vi "Basculas Fabela MultiController.vi"() -> ()   [LabVIEW 2019]
uses:
  <vilib>/Utility/file.llb/Read Delimited Spreadsheet (string).vi
  Subprogramas/Variable global de carga.vi
  <vilib>/Utility/file.llb/Write Delimited Spreadsheet (string).vi
  <vilib>/Utility/error.llb/Error Cluster From Error Code.vi
  <vilib>/ErrorRing/Error Ring.xnode
  <vilib>/Plasmionique/MB Master/MB_Master_Serial/MB_Master_Serial.lvclass
panel:
  in  "Secret button":bool
  out "ReportXlsxPath":path=path "C:/Temp/Basculas Fabela MultiController/Documentos/Reporte.txt"
  out "CtrlClusterOld":T1(array[cluster])
  out "CtrlNumberOld":i32
  in  "ConfChange":bool caption="Lectura de controladores"
  out "PythonPath":path=path "C:/Temp/Insagro/Documentos/TXTaXLSX.exe"
  out "ReportPath":path=path "C:/Temp/Basculas Fabela MultiController/Documentos/Reporte.txt"
  out "ComNumberPath":path=path "C:/Temp/Basculas Fabela MultiController/Documentos/ComNumber.txt"
  out "ComConfigPath":path=path "C:/Temp/Basculas Fabela MultiController/Documentos/ComConfig.txt"
  out "TxtPath":path=path "C:/Temp/Basculas Fabela MultiController/Documentos/Recetas.txt"
  out "Tabs":enum32{"Home", "Main", "Setup"}(tab)=enum."Setup"
  in  "Controllers Load":T2(array[cluster])=[{"ControlerNum"="Controlador 1", "Recipe"="", "Status"=9868950}] caption="Controladores"
  in  "Carga total":bool
  out "Main Load":enum32{"No load", "Load"}(tab)
  out "Ring 2":u16(ring)
  in  "Read":bool caption="Lectura de controladores"
  out "Loading Text":string
  out "TABLA DE RECETAS":string[][](table)
  in  "SecretAnimationCtrl":i32=1 caption="Selección de animación secreta" min=1
  in  "Array CtrlCluster":T1(array[cluster])=[{"Control#"="Control 1", "Com"=""}]
  in  "CtrlNumber":i32=1 caption="Número de controladores" min=1
  in  "Boton Guardar Cambios":bool
  in  "Settings Nav Button":bool=TRUE
  in  "Recetas Nav Button":bool
  in  "Home Nav Button":bool
  # "Seleccione en cada pantalla la fórmula que desee servir"
  # "Peso Objetivo"
  # "Número de Fórmula"
  # "Peso Servido"
  # "Tolva 1"
  # "Tolva 2"
  # "Tolva 3"
  # "Tolva 4"
  # "Indicador Báscula Sirviendo"
  # "Botón Ajuste Manual"
  # "Indicador Falta Material"
  # "FORMULA SELECCIONADA"
  # "CONFIGURACION DE COMUNICACION"
  # "Seleccione los puertos de comunicación"
  # "Controladores"
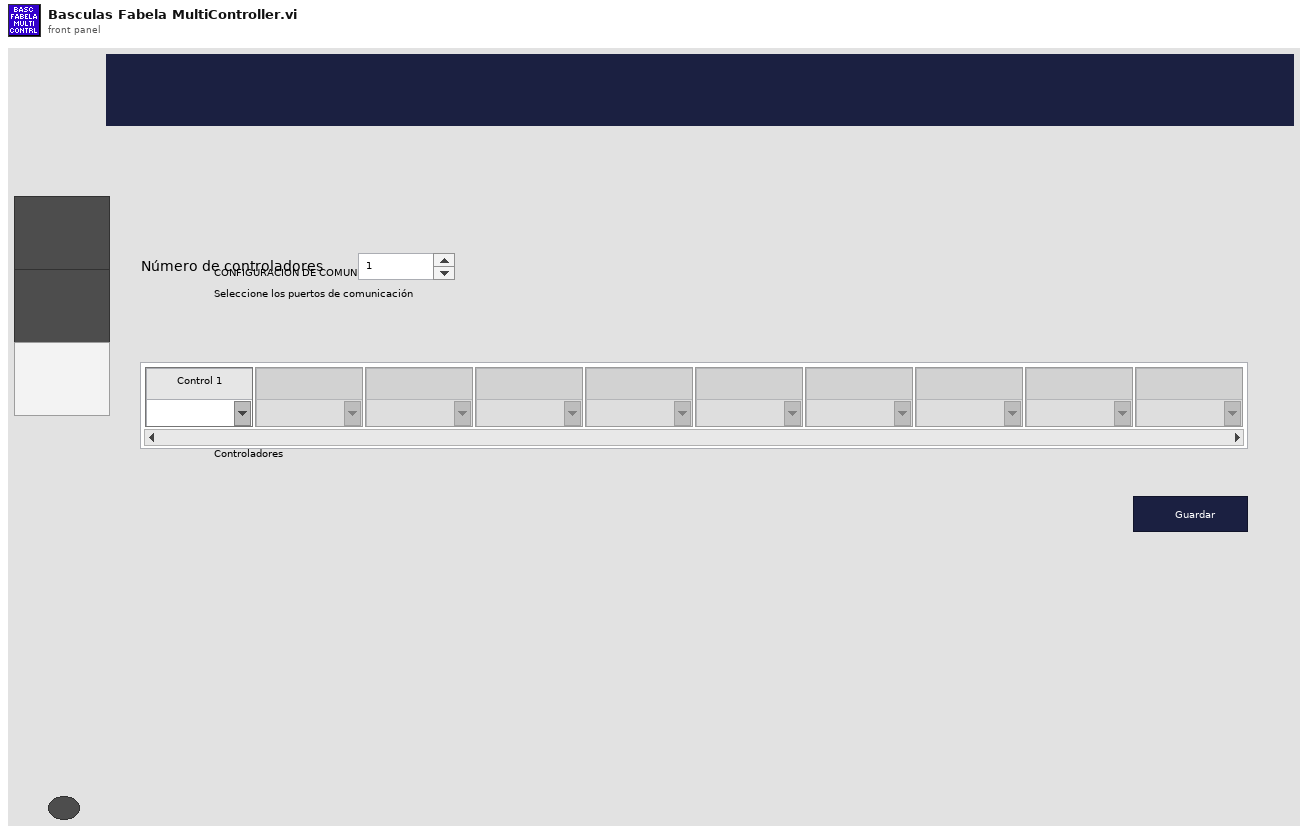
[diagram p1: front panel]
types:
  T1 = cluster{"Control#":string, "Com":refnum<visa-resource-name>}[]
  T2 = cluster{"ControlerNum":string, "Recipe":string, "Status":u32}[]
  T3 = enum8{"Enabled", "Disabled", "Disabled and Grayed Out"}
  T4 = cluster{"Control#":string, "Com":refnum<visa-resource-name>}
  T5 = cluster{"ControlerNum":string, "Recipe":string, "Status":u32}
  T6 = typedef "Control 2.ctl" = refnum<class "MB_Master_Serial.lvclass">[]
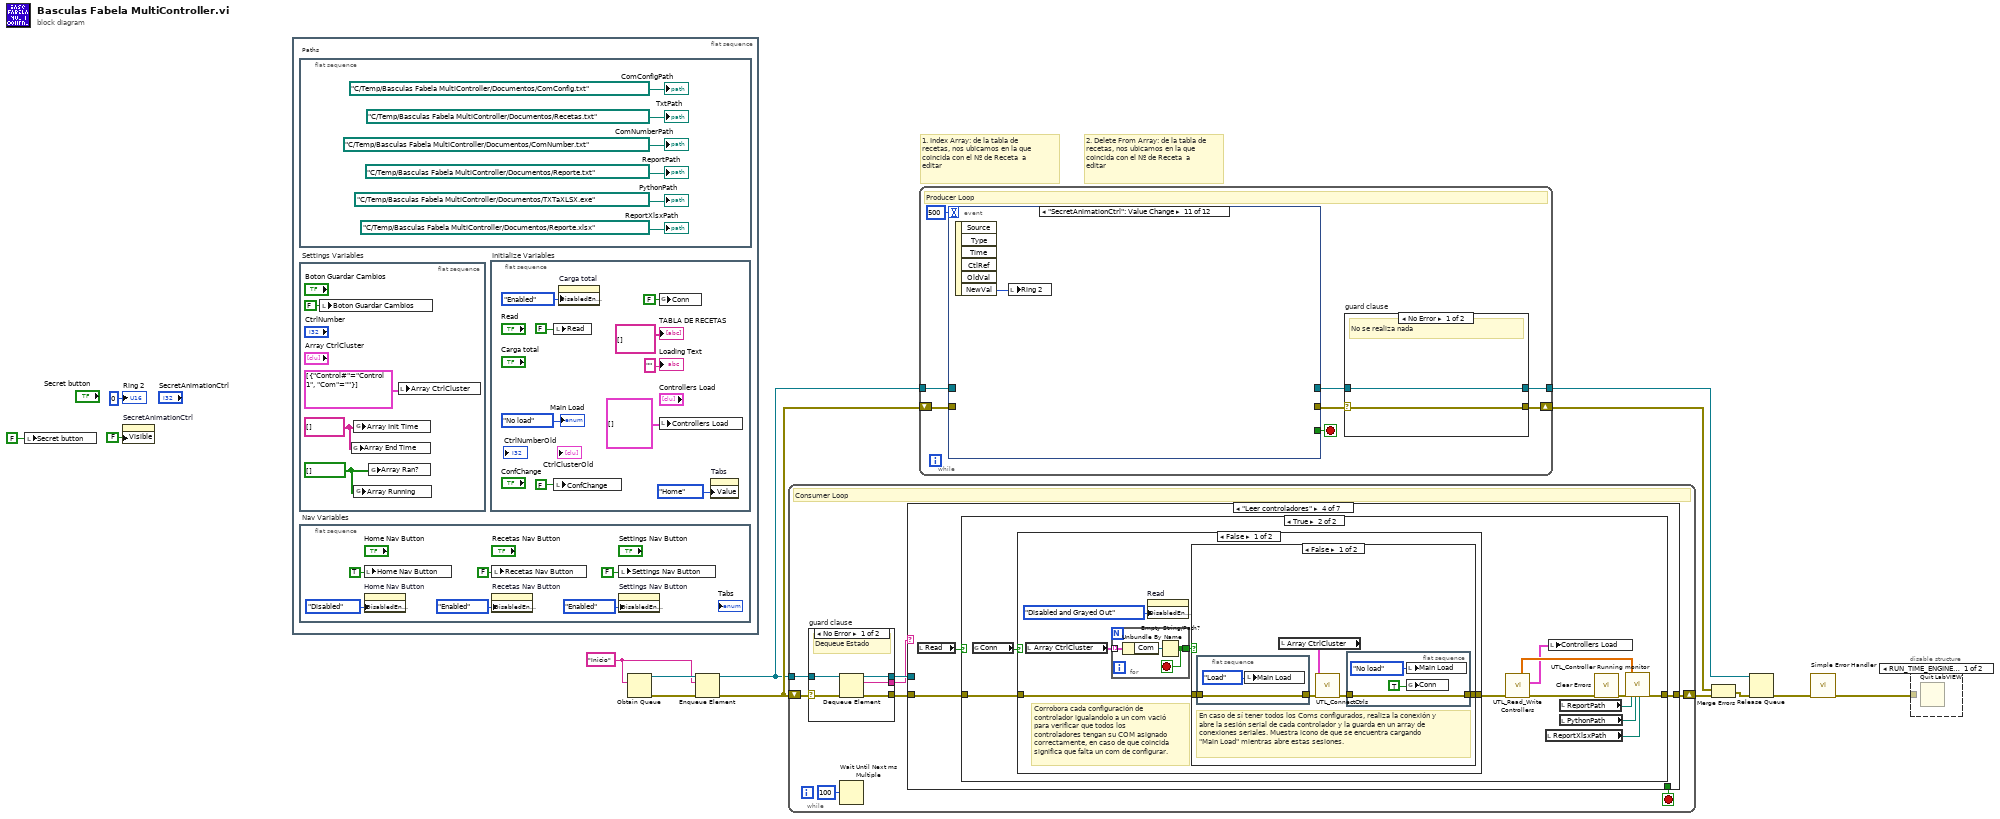
[diagram p0: block diagram]
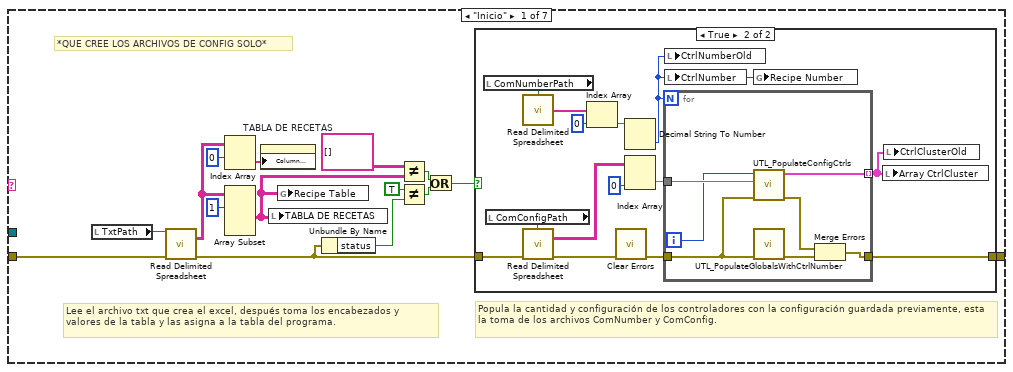
[diagram p2: hidden frame]
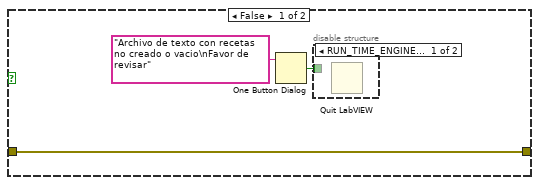
[diagram p3: hidden frame]
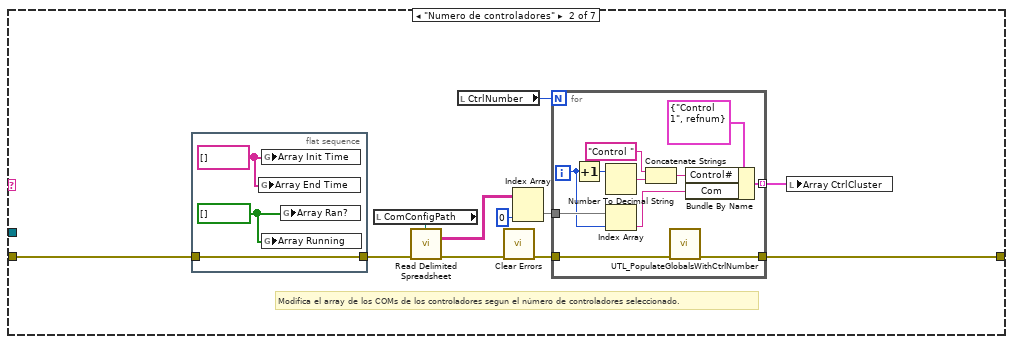
[diagram p5: hidden frame]
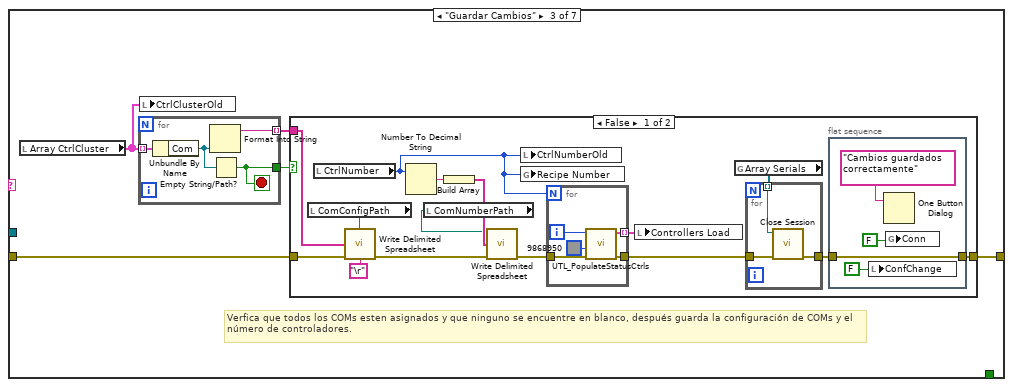
[diagram p6: hidden frame]
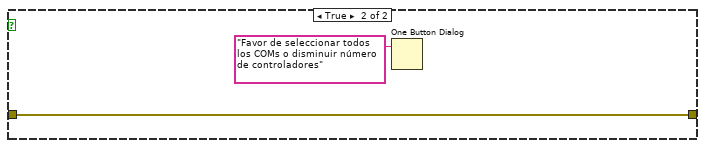
[diagram p7: hidden frame]
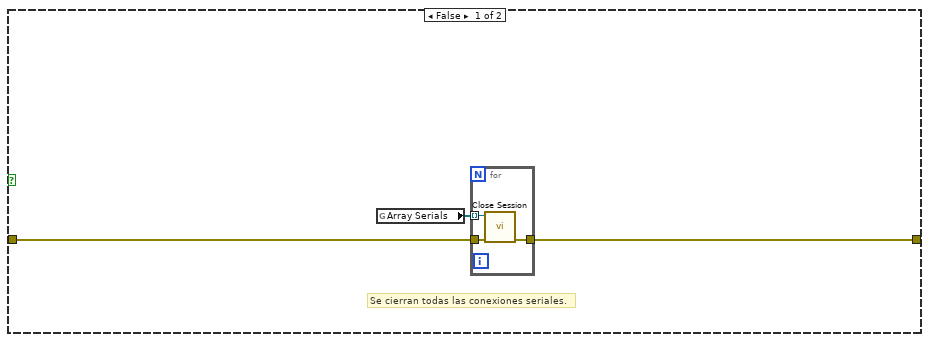
[diagram p8: hidden frame]
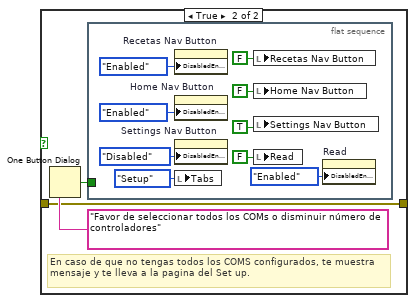
[diagram p9: hidden frame]
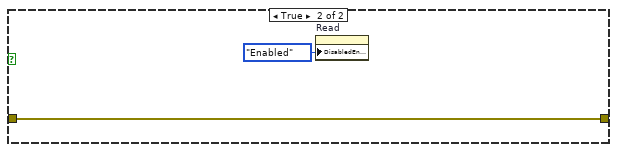
[diagram p10: hidden frame]
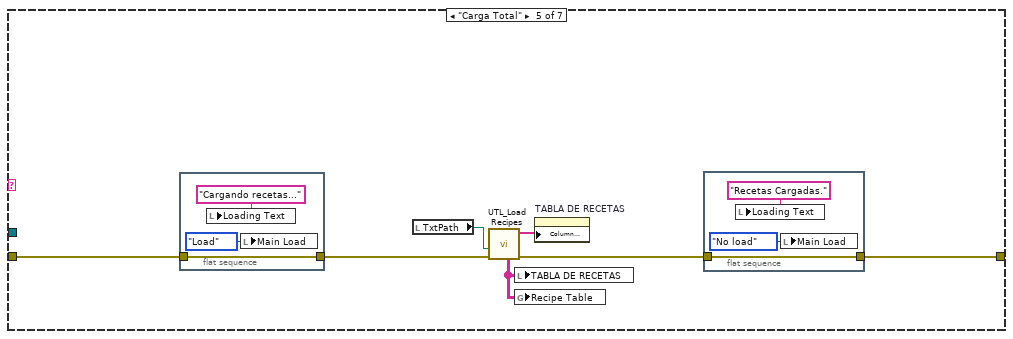
[diagram p11: hidden frame]
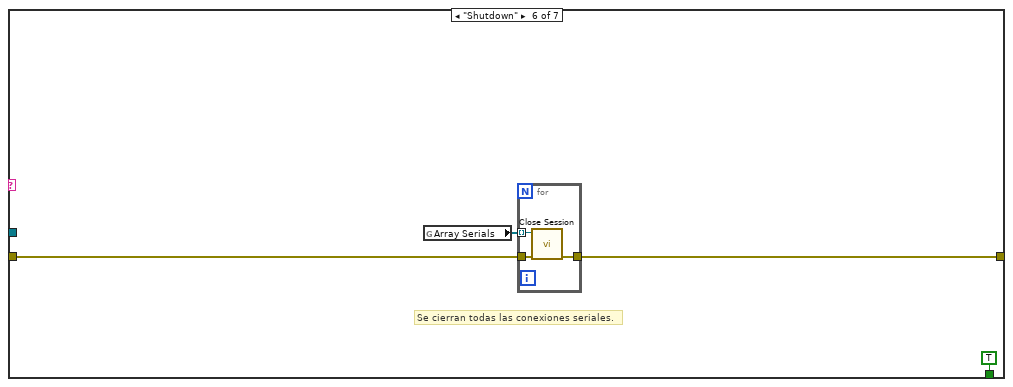
[diagram p12: hidden frame]
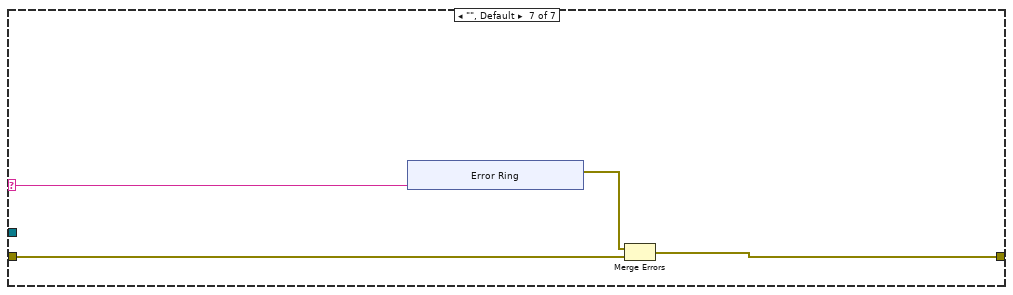
[diagram p13: hidden frame]
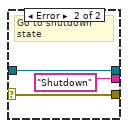
[diagram p14: hidden frame]
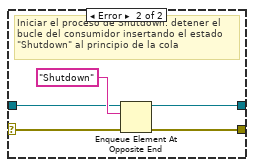
[diagram p15: hidden frame]
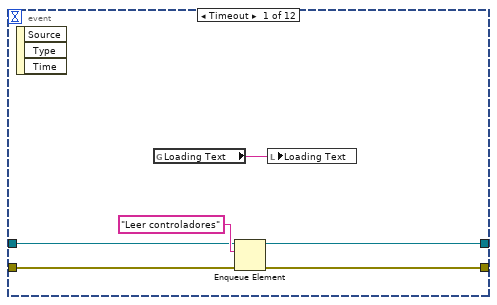
[diagram p16: hidden frame]
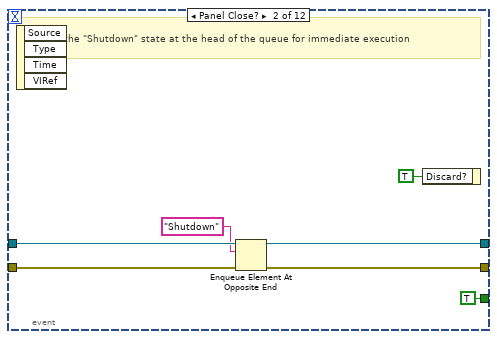
[diagram p17: hidden frame]
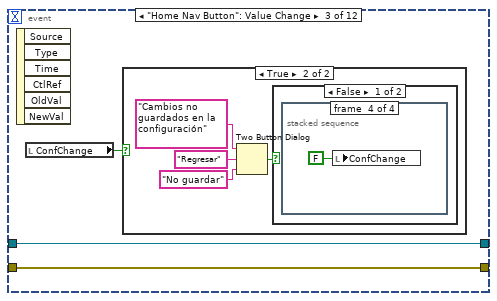
[diagram p18: hidden frame]
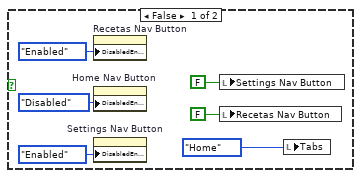
[diagram p19: hidden frame]
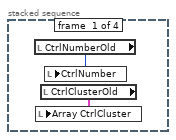
[diagram p20: hidden frame]
diagram:
  w5 = "Inicio"
  # "2. Delete From Array: de la tabla de recetas, nos ubicamos en la que coincida con el Nº de Receta  a editar"
  # "1. Index Array: de la tabla de recetas, nos ubicamos en la que coincida con el Nº de Receta  a editar"
  n1 = local write "Secret button"(FALSE ("Secret button")) -> ()
  n2 = property on="SecretAnimationCtrl" class="DigNum (strict)"("Visible"=FALSE) -> ()  [unwired: 2 in, 2 out]
  n3 = flat-sequence {
    frame #0 {
      # "Initialize Variables"
      # "Nav Variables"
      # "Paths"
      # "Settings Variables"
      n4 = flat-sequence {
        frame #0 {
          "TxtPath" <- path "C:/Temp/Basculas Fabela MultiController/Documentos/Recetas.txt" ("name or relative path")
          "ComConfigPath" <- path "C:/Temp/Basculas Fabela MultiController/Documentos/ComConfig.txt" ("name or relative path")
          "ComNumberPath" <- path "C:/Temp/Basculas Fabela MultiController/Documentos/ComNumber.txt" ("name or relative path")
          "ReportPath" <- path "C:/Temp/Basculas Fabela MultiController/Documentos/Reporte.txt" ("name or relative path")
          "PythonPath" <- path "C:/Temp/Basculas Fabela MultiController/Documentos/TXTaXLSX.exe" ("name or relative path")
          "ReportXlsxPath" <- path "C:/Temp/Basculas Fabela MultiController/Documentos/Reporte.xlsx" ("name or relative path")
        }
      }
      n5 = flat-sequence {
        frame #0 {
          w38 = bool[] [] ("Array Ran?")
          w37 = string[] [] ("Array Init Time")
          n6 = local write "Boton Guardar Cambios"(FALSE ("Boton Iniciar programa")) -> ()
          n7 = global write "Variable global de carga.vi" "Array End Time"(w37) -> ()
          n8 = global write "Variable global de carga.vi" "Array Init Time"(w37) -> ()
          n9 = global write "Variable global de carga.vi" "Array Running"(w38) -> ()
          n10 = global write "Variable global de carga.vi" "Array Ran?"(w38) -> ()
          n11 = local write "Array CtrlCluster"(T1 [{"Control#"="Control 1", "Com"=""}] ("Array CtrlCluster")) -> ()
        }
      }
      n12 = flat-sequence {
        frame #0 {
          n13 = local write "Home Nav Button"(TRUE ("Home Nav Button")) -> ()
          n14 = property on="Home Nav Button" class="Bool (strict)"("DisabledEnum"=T3."Disabled" ("Disabled")) -> ()  [unwired: 2 in, 2 out]
          n15 = local write "Recetas Nav Button"(FALSE ("Recetas Nav Button")) -> ()
          n16 = property on="Recetas Nav Button" class="Bool (strict)"("DisabledEnum"=T3."Enabled" ("Disabled")) -> ()  [unwired: 2 in, 2 out]
          n17 = local write "Settings Nav Button"(FALSE ("Settings Nav Button")) -> ()
          n18 = property on="Settings Nav Button" class="Bool (strict)"("DisabledEnum"=T3."Enabled" ("Disabled")) -> ()  [unwired: 2 in, 2 out]
        }
      }
      n19 = flat-sequence {
        frame #0 {
          n20 = local write "Read"(FALSE ("Read")) -> ()
          n21 = local write "ConfChange"(FALSE ("ConfChange")) -> ()
          n22 = property on="Carga total" class="Bool (strict)"("DisabledEnum"=T3."Enabled" ("Disabled")) -> ()  [unwired: 2 in, 2 out]
          n23 = global write "Variable global de carga.vi" "Conn"(FALSE ("Conn")) -> ()
          n24 = local write "Controllers Load"(T2 [] ("Controllers Load")) -> ()
          n25 = property on="Tabs" class="TabCtl (strict)"("Value"=enum32{"Home", "Main", "Setup"}."Home" ("Tab Control")) -> ()  [unwired: 2 in, 2 out]
          "Main Load" <- enum32{"No load", "Load"}."No load" ("Load C1")
          "TABLA DE RECETAS" <- string[][] []
          "Loading Text" <- "" ("Variable de carga")
        }
      }
    }
  }
  n26 = Obtain Queue(element data type=w5) -> (queue out=w14:refnum<queue>, error out=w13:errorcluster)  [unwired: 4 in, 1 out]
  n27 = Enqueue Element(queue=w14, element=w5, error in (no error)=w13) -> (queue out=w8:refnum<queue>, error out=w9:errorcluster)  [unwired: 1 in, 1 out]
  n28 = while {
    shift-right: [w40] -> w11
    shift-left: w9 -> [w47]
    tunnel: w8 -> [w42]
    stop <- w43 stop-if-true
    # "Consumer Loop"
    n29 = case "guard clause" shown="No Error" w47 {
      selector: w47 -> [w237 w240]
      tunnel: [w236 "Shutdown"] -> w41
      tunnel: [w235 w238] -> w46
      tunnel: [w234 w240] -> w45
      tunnel: w42 -> [w233 w238]
      frame No Error {
        # "Dequeue Estado"
        n30 = Dequeue Element(queue=w233, error in (no error)=w237) -> (queue out=w235:refnum<queue>, element=w236:string, error out=w234:errorcluster)  [unwired: 1 in, 1 out]
      }
      frame Error {
        # "Go to shutdown state"
      }
    }
    n31 = Wait Until Next ms Multiple(millisecond multiple=u32 100) -> ()  [unwired: 1 out]
    n32 = case shown="\"Leer controladores\"" w41 {
      selector: w41 -> [_ _ _ _ _ _ w225]
      tunnel: w46 -> [_ _ _ _ _ _ _]
      tunnel: w45 -> [w53 w90 w113 w151 w207 w217 w224]
      tunnel: [_ _ _ _ _ TRUE _] -> w43
      tunnel: [w51 w87 w116 w150 w204 w216 w222] -> w40
      frame "Inicio" {
        # "*QUE CREE LOS ARCHIVOS DE CONFIG SOLO*"
        # "Popula la cantidad y configuración de los controladores con la configuración guardada previamente, esta la toma de los archivos ComNumber y ComConfig."
        # "Lee el archivo txt que crea el excel, después toma los encabezados y valores de la tabla y las asigna a la tabla del programa."
        n33 = local read "TxtPath"() -> (w56:path)
        n34 = call-poly <vilib>:"Read Delimited Spreadsheet.vi"("file path (dialog if empty)"=w56, "error in (no error)"=w53) -> ("all rows"=w61:string[][], "error out"=w52:errorcluster)  [unwired: 8 in, 4 out]
        n35 = Index Array(array=w61, index (row)=0) -> (element=w62:string[])  [unwired: 1 in]
        n36 = Array Subset(array=w61, index (row)=1 ("index")) -> (w50:string[][])  [unwired: 3 in]
        n37 = property on="TABLA DE RECETAS" class="Tbl (strict)"("Column Headers[]"=w62) -> ()  [unwired: 2 in, 2 out]
        n38 = local write "TABLA DE RECETAS"(w50) -> ()
        n39 = global write "Variable global de carga.vi" "Recipe Table"(w50) -> ()
        n40 = Unbundle By Name(w52) -> ("status"=w59:bool)
        n41 = Not Equal?(x=string[][] [], y=w50) -> (x != y?=w58:bool)
        n42 = Not Equal?(x=TRUE, y=w59) -> (x != y?=w60:bool)
        n43 = Or(x=w58, y=w60) -> (x .or. y?=w57:bool)
        n44 = case shown="True" w57 {
          tunnel: w52 -> [w63 w75]
          tunnel: [w63 w68] -> w51
          frame False {
            n45 = One Button Dialog(message="Archivo de texto con recetas no creado o vacio\nFavor de revisar") -> (true=w64:bool)  [unwired: 1 in]
            n46 = disable-structure shown="RUN_TIME_ENGINE==True" {
              disable-tunnel: w64 -> [_ _]
              frame condition #0 {
                n47 = Quit LabVIEW() -> ()  [unwired: 1 in]
              }
              frame condition #1 (active) {
              }
            }
          }
          frame True {
            n48 = local read "ComNumberPath"() -> (w74:path)
            n49 = local read "ComConfigPath"() -> (w76:path)
            n50 = call-poly <vilib>:"Read Delimited Spreadsheet.vi"("file path (dialog if empty)"=w74) -> ("first row"=w73:string[])  [unwired: 9 in, 5 out]
            n51 = call-poly <vilib>:"Read Delimited Spreadsheet.vi"("file path (dialog if empty)"=w76, "error in (no error)"=w75) -> ("all rows"=w79:string[][], "error out"=w77:errorcluster)  [unwired: 8 in, 4 out]
            n52 = Index Array(array=w73, index=0 ("disabled index (col)")) -> (element=w72:string)
            n53 = call <vilib>:"Clear Errors.vi"("error in (no error)"=w77) -> ("error out"=w69:errorcluster)  [unwired: 5 in, 1 out]
            n54 = Decimal String To Number(string=w72) -> (number=w66:i32)  [unwired: 2 in, 1 out]
            n55 = Index Array(array=w79, index (col)=0 ("disabled index (col)")) -> (element=w70:string[])  [unwired: 1 in]
            n56 = for {
              N: w66 -> [_]
              tunnel: w70 -> [w86]
              tunnel: w69 -> [w82]
              tunnel: [w83] -> w68
              tunnel: [w85] -> w67 mode=indexing
              i -> [w81]
              n57 = call "UTL_PopulateConfigCtrls.vi"("error in (no error)"=w82, "ComConfig"=w86, "ComNum"=w81) -> ("error out"=w80:errorcluster, "Array Cluster"=w85:T4)  [unwired: 7 in]
              n58 = call "UTL_PopulateGlobalsWithCtrlNumber.vi"("error in (no error)"=w82) -> ("error out"=w84:errorcluster)  [unwired: 10 in]
              n59 = Merge Errors(w80, w84) -> (w83:errorcluster)
            }
            n60 = local write "CtrlNumberOld"(w66) -> ()
            n61 = local write "CtrlNumber"(w66) -> ()
            n62 = global write "Variable global de carga.vi" "Recipe Number"(w66) -> ()
            n63 = local write "Array CtrlCluster"(w67) -> ()
            n64 = local write "CtrlClusterOld"(w67) -> ()
          }
        }
      }
      frame "Numero de controladores" {
        # "Modifica el array de los COMs de los controladores segun el número de controladores seleccionado."
        n65 = flat-sequence {
          tunnel: w90 -> [w98]
          tunnel: [w98] -> w89
          frame #0 {
            w100 = bool[] [] ("Array Ran?")
            w99 = string[] [] ("Array Init Time")
            n66 = global write "Variable global de carga.vi" "Array End Time"(w99) -> ()
            n67 = global write "Variable global de carga.vi" "Array Init Time"(w99) -> ()
            n68 = global write "Variable global de carga.vi" "Array Running"(w100) -> ()
            n69 = global write "Variable global de carga.vi" "Array Ran?"(w100) -> ()
          }
        }
        n70 = local read "ComConfigPath"() -> (w95:path)
        n71 = call-poly <vilib>:"Read Delimited Spreadsheet.vi"("file path (dialog if empty)"=w95, "error in (no error)"=w89) -> ("all rows"=w97:string[][], "error out"=w96:errorcluster)  [unwired: 8 in, 4 out]
        n72 = local read "CtrlNumber"() -> (w91:i32)
        n73 = call <vilib>:"Clear Errors.vi"("error in (no error)"=w96) -> ("error out"=w88:errorcluster)  [unwired: 5 in, 1 out]
        n74 = Index Array(array=w97, index (col)=0 ("disabled index (col)")) -> (element=w94:string[])  [unwired: 1 in]
        n75 = for {
          N: w91 -> [_]
          tunnel: w94 -> [w105]
          tunnel: [w106] -> w93 mode=indexing
          tunnel: w88 -> [w102]
          tunnel: [w101] -> w87
          i -> [w104]
          n76 = Increment(x=w104) -> (x+1=w107:i32)
          n77 = Number To Decimal String(number=w107) -> (decimal integer string=w111:string)  [unwired: 1 in]
          n78 = Index Array(array=w105, index=w104) -> (element=w103:string)
          n79 = Concatenate Strings("Control " ("Control#"), w111) -> (w110:string)
          n80 = call "UTL_PopulateGlobalsWithCtrlNumber.vi"("error in (no error)"=w102) -> ("error out"=w101:errorcluster)  [unwired: 10 in]
          n81 = Bundle By Name(cluster=T4 {"Control#"="Control 1", "Com"=""} ("CtrlClust"), "Control#"=w110, "Com"=w103) -> (w106:T4)
        }
        n82 = local write "Array CtrlCluster"(w93) -> ()
      }
      frame "Guardar Cambios" {
        # "Verfica que todos los COMs esten asignados y que ninguno se encuentre en blanco, después guarda la configuración de COMs y el número de controladores."
        n83 = local read "Array CtrlCluster"() -> (w112:T1)
        n84 = for {
          tunnel: [w146] -> w114
          tunnel: [w149] -> w115 mode=indexing
          tunnel: w112 -> [w148] mode=indexing
          stop <- w146 stop-if-true
          n85 = Unbundle By Name(w148) -> ("Com"=w147:refnum<visa-resource-name>)
          n86 = Format Into String(w147) -> (resulting string=w149:string)  [unwired: 3 in, 1 out]
          n87 = Empty String/Path?(string/path=w147) -> (empty?=w146:bool)
        }
        n88 = local write "CtrlClusterOld"(w112) -> ()
        n89 = case shown="False" w114 {
          tunnel: w115 -> [w130 _]
          tunnel: [w126 w144] -> w116
          tunnel: w113 -> [w129 w144]
          frame False {
            n90 = local read "ComConfigPath"() -> (w128:path)
            n91 = local read "CtrlNumber"() -> (w117:i32)
            n92 = call-poly <vilib>:"Write Delimited Spreadsheet.vi"("file path (dialog if empty)"=w128, "1D data"=w130, "error in (no error)"=w129, "delimiter (\\t)"="\r") -> ("error out"=w122:errorcluster)  [unwired: 10 in, 1 out]
            n93 = Number To Decimal String(number=w117) -> (decimal integer string=w124:string)  [unwired: 1 in]
            n94 = local read "ComNumberPath"() -> (w121:path)
            n95 = Build Array(w124) -> (w123:string[])
            n96 = call-poly <vilib>:"Write Delimited Spreadsheet.vi"("file path (dialog if empty)"=w121, "1D data"=w123, "error in (no error)"=w122) -> ("error out"=w120:errorcluster)  [unwired: 11 in, 1 out]
            n97 = local write "CtrlNumberOld"(w117) -> ()
            n98 = global write "Variable global de carga.vi" "Recipe Number"(w117) -> ()
            n99 = for {
              N: w117 -> [_]
              tunnel: w120 -> [w136]
              tunnel: [w135] -> w119
              tunnel: [w132] -> w118 mode=indexing
              i -> [w133]
              n100 = call "UTL_PopulateStatusCtrls.vi"("error in (no error)"=w136, "Status"=u32 9868950, "ComNum"=w133) -> ("error out"=w135:errorcluster, "output cluster"=w132:T5)  [unwired: 7 in]
            }
            n101 = local write "Controllers Load"(w118) -> ()
            n102 = global read "Variable global de carga.vi" "Array Serials"() -> (w125:T6)
            n103 = for {
              tunnel: [w143] -> w127
              tunnel: w119 -> [w142]
              tunnel: w125 -> [w141] mode=indexing
              n104 = call-dynamic "Close Session.vi"("error in (no error)"=w142, "MB_Serial session"=w141) -> ("error out"=w143:errorcluster)  [unwired: 9 in]
            }
            n105 = flat-sequence {
              tunnel: w127 -> [w140]
              tunnel: [w140] -> w126
              frame #0 {
                n106 = local write "ConfChange"(FALSE ("ConfChange")) -> ()
                n107 = One Button Dialog(message="Cambios guardados correctamente") -> ()  [unwired: 1 in, 1 out]
                n108 = global write "Variable global de carga.vi" "Conn"(FALSE ("Conn")) -> ()
              }
            }
          }
          frame True {
            n109 = One Button Dialog(message="Favor de seleccionar todos los COMs o disminuir número de controladores") -> ()  [unwired: 1 in, 1 out]
          }
        }
      }
      frame "Leer controladores" {
        n110 = local read "Read"() -> (w152:bool)
        n111 = case shown="True" w152 {
          tunnel: [w153 w169] -> w150
          tunnel: w151 -> [w154 w163]
          frame False {
            # "Se cierran todas las conexiones seriales."
            n112 = global read "Variable global de carga.vi" "Array Serials"() -> (w155:T6)
            n113 = for {
              tunnel: [w158] -> w153
              tunnel: w154 -> [w157]
              tunnel: w155 -> [w156] mode=indexing
              n114 = call-dynamic "Close Session.vi"("error in (no error)"=w157, "MB_Serial session"=w156) -> ("error out"=w158:errorcluster)  [unwired: 9 in]
            }
          }
          frame True {
            n115 = global read "Variable global de carga.vi" "Conn"() -> (w165:bool)
            n116 = case shown="False" w165 {
              tunnel: [w174 w201] -> w164
              tunnel: w163 -> [w171 w201]
              frame False {
                # "Corrobora cada configuración de controlador igualandolo a un com vació para verificar que todos los controladores tengan su COM asignado correctamente, en caso de que coincida significa que falta un com de configurar."
                n117 = local read "Array CtrlCluster"() -> (w172:T1)
                n118 = for {
                  tunnel: [w175] -> w173
                  tunnel: w172 -> [w177] mode=indexing
                  stop <- w175 stop-if-true
                  n119 = Unbundle By Name(w177) -> ("Com"=w176:refnum<visa-resource-name>)
                  n120 = Empty String/Path?(string/path=w176) -> (empty?=w175:bool)
                }
                n121 = property on="Read" class="Bool (strict)"("DisabledEnum"=T3."Disabled and Grayed Out" ("Disabled")) -> ()  [unwired: 2 in, 2 out]
                n122 = case shown="False" w173 {
                  tunnel: [w182 w188] -> w174
                  tunnel: w171 -> [w178 w188]
                  frame False {
                    # "En caso de sí tener todos los Coms configurados, realiza la conexión y abre la sesión serial de cada controlador y la guarda en un array de conexiones seriales. Muestra icono de que se encuentra cargando \"Main Load\" mientras abre estas sesiones."
                    n123 = flat-sequence {
                      tunnel: [w186] -> w179
                      tunnel: w178 -> [w186]
                      frame #0 {
                        n124 = local write "Main Load"(enum32{"No load", "Load"}."Load" ("Load C1")) -> ()
                      }
                    }
                    n125 = local read "Array CtrlCluster"() -> (w180:T1)
                    n126 = call "UTL_ConnectCtrls.vi"("error in (no error)"=w179, "Array CtrlCluster"=w180) -> ("error out"=w181:errorcluster)  [unwired: 9 in]
                    n127 = flat-sequence {
                      tunnel: w181 -> [w184]
                      tunnel: [w184] -> w182
                      frame #0 {
                        n128 = local write "Main Load"(enum32{"No load", "Load"}."No load" ("Load C1")) -> ()
                        n129 = global write "Variable global de carga.vi" "Conn"(TRUE ("Conn")) -> ()
                      }
                    }
                  }
                  frame True {
                    # "En caso de que no tengas todos los COMS configurados, te muestra mensaje y te lleva a la pagina del Set up."
                    n130 = One Button Dialog(message="Favor de seleccionar todos los COMs o disminuir número de controladores") -> (true=w189:bool)  [unwired: 1 in]
                    n131 = flat-sequence {
                      tunnel: w189 -> [_]
                      frame #0 {
                        n132 = property on="Recetas Nav Button" class="Bool (strict)"("DisabledEnum"=T3."Enabled" ("Disabled")) -> ()  [unwired: 2 in, 2 out]
                        n133 = property on="Home Nav Button" class="Bool (strict)"("DisabledEnum"=T3."Enabled" ("Disabled")) -> ()  [unwired: 2 in, 2 out]
                        n134 = property on="Settings Nav Button" class="Bool (strict)"("DisabledEnum"=T3."Disabled" ("Disabled")) -> ()  [unwired: 2 in, 2 out]
                        n135 = local write "Tabs"(enum32{"Home", "Main", "Setup"}."Setup" ("Pagina programa")) -> ()
                        n136 = local write "Recetas Nav Button"(FALSE ("Recetas Nav Button")) -> ()
                        n137 = local write "Home Nav Button"(FALSE ("Settings Nav Button")) -> ()
                        n138 = local write "Settings Nav Button"(TRUE ("Settings Nav Button")) -> ()
                        n139 = local write "Read"(FALSE ("Read")) -> ()
                        n140 = property on="Read" class="Bool (strict)"("DisabledEnum"=T3."Enabled" ("Disabled")) -> ()  [unwired: 2 in, 2 out]
                      }
                    }
                  }
                }
              }
              frame True {
                n141 = property on="Read" class="Bool (strict)"("DisabledEnum"=T3."Enabled" ("Disabled")) -> ()  [unwired: 2 in, 2 out]
              }
            }
            n142 = call "UTL_Read_Write Controllers.vi"("error in"=w164) -> ("error out"=w168:errorcluster, "StatusCtrl"=w166:T2, "Results"=w167:dbl[][][])  [unwired: 8 in]
            n143 = local read "ReportXlsxPath"() -> (w159:path)
            n144 = local write "Controllers Load"(w166) -> ()
            n145 = local read "ReportPath"() -> (w161:path)
            n146 = local read "PythonPath"() -> (w160:path)
            n147 = call <vilib>:"Clear Errors.vi"("error in (no error)"=w168) -> ("error out"=w162:errorcluster)  [unwired: 5 in, 1 out]
            n148 = call "UTL_Controller Running monitor.vi"("Error In"=w162, "Data"=w167, "ReportPath"=w161, "PyPath"=w160, "ReportXlsxPath"=w159) -> ("Error Out"=w169:errorcluster)  [unwired: 14 in]
          }
        }
      }
      frame "Carga Total" {
        n149 = flat-sequence {
          tunnel: w207 -> [w213]
          tunnel: [w213] -> w208
          frame #0 {
            n150 = local write "Loading Text"("Cargando recetas..." ("Carga texto")) -> ()
            n151 = local write "Main Load"(enum32{"No load", "Load"}."Load" ("Load C1")) -> ()
          }
        }
        n152 = local read "TxtPath"() -> (w206:path)
        n153 = call "UTL_Load Recipes.vi"("Error in"=w208, "Txt Path"=w206) -> ("Error out"=w205:errorcluster, "Headers"=w203:string[], "Sorted 2D table array"=w202:string[][])  [unwired: 7 in]
        n154 = local write "TABLA DE RECETAS"(w202) -> ()
        n155 = global write "Variable global de carga.vi" "Recipe Table"(w202) -> ()
        n156 = property on="TABLA DE RECETAS" class="Tbl (strict)"("Column Headers[]"=w203) -> ()  [unwired: 2 in, 2 out]
        n157 = flat-sequence {
          tunnel: w205 -> [w210]
          tunnel: [w210] -> w204
          frame #0 {
            n158 = local write "Loading Text"("Recetas Cargadas." ("Carga texto")) -> ()
            n159 = local write "Main Load"(enum32{"No load", "Load"}."No load" ("Load C1")) -> ()
          }
        }
      }
      frame "Shutdown" {
        # "Se cierran todas las conexiones seriales."
        # "Stop the Consumer Loop, and signal the Producer Loop to also stop by activating the front-panel \"Stop\" button; use the \"signaling\" version to trigger the event structure"
        n160 = global read "Variable global de carga.vi" "Array Serials"() -> (w215:T6)
        n161 = for {
          tunnel: [w221] -> w216
          tunnel: w217 -> [w220]
          tunnel: w215 -> [w219] mode=indexing
          n162 = call-dynamic "Close Session.vi"("error in (no error)"=w220, "MB_Serial session"=w219) -> ("error out"=w221:errorcluster)  [unwired: 9 in]
        }
      }
      frame "", Default {
        # "Handle unknown states"
        n163 = xnode "Error Ring"("parameter 0"=w225) -> ("error out"=w223:errorcluster)
        n164 = Merge Errors(w223, w224) -> (w222:errorcluster)
      }
    }
  }
  n165 = while {
    shift-right: [w243] -> w7
    shift-left: w9 -> [w247]
    tunnel: w8 -> [w246]
    tunnel: [w244] -> w6
    stop <- w242 stop-if-true
    # "Producer Loop"
    n166 = event shown="[10] \"SecretAnimationCtrl\": Value Change" {
      selector: _ -> [_ _ _ _ _ _ _ _ _ _ _ _]
      dyn-events: _ -> [_ _ _ _ _ _ _ _ _ _ _ _]
      timeout: 500 -> [_ _ _ _ _ _ _ _ _ _ _ _]
      tunnel: [w258 w265 w270 w296 w325 w329 w343 w351 w358 _ _ w374] -> w248
      tunnel: w247 -> [w259 w266 w270 w296 w325 w330 w344 w351 w358 _ _ w375]
      tunnel: w246 -> [w256 w268 w271 w295 w324 w331 w346 w352 w357 _ _ w376]
      tunnel: [_ TRUE _ _ _ _ _ _ _ _ _ _] -> w242
      tunnel: [w257 w263 w271 w295 w324 w328 w342 w352 w357 _ _ w373] -> w245
      event Timeout {
        n167 = event-data() -> ()  [unwired: 1 in, 3 out]
        n168 = global read "Variable global de carga.vi" "Loading Text"() -> (w261:string)
        n169 = Enqueue Element(queue=w256, element="Leer controladores", error in (no error)=w259) -> (queue out=w257:refnum<queue>, error out=w258:errorcluster)  [unwired: 1 in, 1 out]
        n170 = local write "Loading Text"(w261) -> ()
      }
      event Panel Close? {
        # "Enqueue the \"Shutdown\" state at the head of the queue for immediate execution"
        n171 = event-data() -> ()  [unwired: 1 in, 4 out]
        n172 = Enqueue Element At Opposite End(queue=w268, element="Shutdown", error in (no error)=w266) -> (queue out=w263:refnum<queue>, error out=w265:errorcluster)  [unwired: 1 in, 1 out]
        n173 = event-data("Discard?"=TRUE) -> ()  [unwired: 1 in, 1 out]
      }
      event "Home Nav Button": Value Change {
        n174 = event-data() -> ()  [unwired: 1 in, 6 out]
        n175 = local read "ConfChange"() -> (w269:bool)
        n176 = case shown="True" w269 {
          frame False {
            n177 = property on="Recetas Nav Button" class="Bool (strict)"("DisabledEnum"=T3."Enabled" ("Disabled")) -> ()  [unwired: 2 in, 2 out]
            n178 = property on="Home Nav Button" class="Bool (strict)"("DisabledEnum"=T3."Disabled" ("Disabled")) -> ()  [unwired: 2 in, 2 out]
            n179 = property on="Settings Nav Button" class="Bool (strict)"("DisabledEnum"=T3."Enabled" ("Disabled")) -> ()  [unwired: 2 in, 2 out]
            n180 = local write "Settings Nav Button"(FALSE ("Settings Nav Button")) -> ()
            n181 = local write "Recetas Nav Button"(FALSE ("Recetas Nav Button")) -> ()
            n182 = local write "Tabs"(enum32{"Home", "Main", "Setup"}."Home" ("Pagina programa")) -> ()
          }
          frame True {
            n183 = Two Button Dialog(message="Cambios no guardados en la configuración", 1:"No guardar" ("F button name (\"Cancel\")"), 2:"Regresar" ("T button name (\"OK\")")) -> (T button?=w278:bool)
            n184 = case shown="False" w278 {
              frame False {
                n185 = stacked-sequence {
                  frame #0 {
                    n186 = local read "CtrlNumberOld"() -> (w282:i32)
                    n187 = local read "CtrlClusterOld"() -> (w283:T1)
                    n188 = local write "Array CtrlCluster"(w283) -> ()
                    n189 = local write "CtrlNumber"(w282) -> ()
                  }
                  frame #1 {
                    w285 = T3."Enabled" ("Disabled")
                    n190 = property on="Settings Nav Button" class="Bool (strict)"("DisabledEnum"=w285) -> ()  [unwired: 2 in, 2 out]
                    n191 = property on="Recetas Nav Button" class="Bool (strict)"("DisabledEnum"=w285) -> ()  [unwired: 2 in, 2 out]
                    n192 = property on="Home Nav Button" class="Bool (strict)"("DisabledEnum"=T3."Disabled" ("Disabled")) -> ()  [unwired: 2 in, 2 out]
                  }
                  frame #2 {
                    n193 = local write "Settings Nav Button"(FALSE ("Settings Nav Button")) -> ()
                    n194 = local write "Recetas Nav Button"(FALSE ("Recetas Nav Button")) -> ()
                    n195 = local write "Tabs"(enum32{"Home", "Main", "Setup"}."Home" ("Pagina programa")) -> ()
                  }
                  frame #3 {
                    n196 = local write "ConfChange"(FALSE ("ConfChange")) -> ()
                  }
                }
              }
              frame True {
                n197 = local write "Recetas Nav Button"(FALSE ("Recetas Nav Button")) -> ()
                n198 = local write "Home Nav Button"(FALSE ("Settings Nav Button")) -> ()
                n199 = local write "Settings Nav Button"(TRUE ("Settings Nav Button")) -> ()
                n200 = local write "Tabs"(enum32{"Home", "Main", "Setup"}."Setup" ("Pagina programa")) -> ()
              }
            }
          }
        }
      }
      event "Recetas Nav Button": Value Change {
        n201 = event-data() -> ()  [unwired: 1 in, 6 out]
        n202 = local read "ConfChange"() -> (w294:bool)
        n203 = case shown="True" w294 {
          frame False {
            n204 = property on="Recetas Nav Button" class="Bool (strict)"("DisabledEnum"=T3."Disabled" ("Disabled")) -> ()  [unwired: 2 in, 2 out]
            n205 = property on="Home Nav Button" class="Bool (strict)"("DisabledEnum"=T3."Enabled" ("Disabled")) -> ()  [unwired: 2 in, 2 out]
            n206 = property on="Settings Nav Button" class="Bool (strict)"("DisabledEnum"=T3."Enabled" ("Disabled")) -> ()  [unwired: 2 in, 2 out]
            n207 = local write "Home Nav Button"(FALSE ("Recetas Nav Button")) -> ()
            n208 = local write "Settings Nav Button"(FALSE ("Settings Nav Button")) -> ()
            n209 = local write "Tabs"(enum32{"Home", "Main", "Setup"}."Main" ("Pagina programa")) -> ()
          }
          frame True {
            n210 = Two Button Dialog(message="Cambios no guardados en la configuración", 1:"No guardar" ("F button name (\"Cancel\")"), 2:"Regresar" ("T button name (\"OK\")")) -> (T button?=w306:bool)
            n211 = case shown="False" w306 {
              frame False {
                n212 = stacked-sequence {
                  frame #0 {
                    n213 = local read "CtrlNumberOld"() -> (w307:i32)
                    n214 = local read "CtrlClusterOld"() -> (w308:T1)
                    n215 = local write "Array CtrlCluster"(w308) -> ()
                    n216 = local write "CtrlNumber"(w307) -> ()
                  }
                  frame #1 {
                    w310 = T3."Enabled" ("Disabled")
                    n217 = property on="Recetas Nav Button" class="Bool (strict)"("DisabledEnum"=T3."Disabled" ("Disabled")) -> ()  [unwired: 2 in, 2 out]
                    n218 = property on="Home Nav Button" class="Bool (strict)"("DisabledEnum"=w310) -> ()  [unwired: 2 in, 2 out]
                    n219 = property on="Settings Nav Button" class="Bool (strict)"("DisabledEnum"=w310) -> ()  [unwired: 2 in, 2 out]
                  }
                  frame #2 {
                    n220 = local write "Home Nav Button"(FALSE ("Recetas Nav Button")) -> ()
                    n221 = local write "Settings Nav Button"(FALSE ("Settings Nav Button")) -> ()
                    n222 = local write "Tabs"(enum32{"Home", "Main", "Setup"}."Main" ("Pagina programa")) -> ()
                  }
                  frame #3 {
                    n223 = local write "ConfChange"(FALSE ("ConfChange")) -> ()
                  }
                }
              }
              frame True {
                n224 = local write "Recetas Nav Button"(FALSE ("Recetas Nav Button")) -> ()
                n225 = local write "Home Nav Button"(FALSE ("Settings Nav Button")) -> ()
                n226 = local write "Settings Nav Button"(TRUE ("Settings Nav Button")) -> ()
                n227 = local write "Tabs"(enum32{"Home", "Main", "Setup"}."Setup" ("Pagina programa")) -> ()
              }
            }
          }
        }
      }
      event "Settings Nav Button": Value Change {
        n228 = event-data() -> ()  [unwired: 1 in, 6 out]
        n229 = property on="Recetas Nav Button" class="Bool (strict)"("DisabledEnum"=T3."Enabled" ("Disabled")) -> ()  [unwired: 2 in, 2 out]
        n230 = property on="Home Nav Button" class="Bool (strict)"("DisabledEnum"=T3."Enabled" ("Disabled")) -> ()  [unwired: 2 in, 2 out]
        n231 = property on="Settings Nav Button" class="Bool (strict)"("DisabledEnum"=T3."Disabled" ("Disabled")) -> ()  [unwired: 2 in, 2 out]
        n232 = local write "Home Nav Button"(FALSE ("Recetas Nav Button")) -> ()
        n233 = local write "Recetas Nav Button"(FALSE ("Recetas Nav Button")) -> ()
        n234 = local write "Tabs"(enum32{"Home", "Main", "Setup"}."Setup" ("Pagina programa")) -> ()
      }
      event "Carga total": Value Change {
        n235 = event-data() -> ("NewVal"=w327:bool)  [unwired: 1 in, 5 out]
        n236 = case shown="True" w327 {
          tunnel: w331 -> [w333 w338]
          tunnel: w330 -> [w332 w336]
          tunnel: [w332 w335] -> w329
          tunnel: [w333 w334] -> w328
          frame False {
          }
          frame True {
            n237 = Enqueue Element(queue=w338, element="Carga Total", error in (no error)=w336) -> (queue out=w334:refnum<queue>, error out=w335:errorcluster)  [unwired: 1 in, 1 out]
          }
        }
      }
      event "CtrlNumber": Value Change {
        n238 = event-data() -> ()  [unwired: 1 in, 6 out]
        n239 = local read "CtrlNumberOld"() -> (w340:i32)
        n240 = local read "CtrlNumber"() -> (w339:i32)
        n241 = Not Equal?(x=w340, y=w339) -> (x != y?=w341:bool)
        n242 = case shown="False" w341 {
          frame False {
            n243 = local write "ConfChange"(FALSE ("ConfChange")) -> ()
          }
          frame True {
            n244 = local write "ConfChange"(TRUE ("ConfChange")) -> ()
          }
        }
        n245 = Enqueue Element(queue=w346, element="Numero de controladores", error in (no error)=w344) -> (queue out=w342:refnum<queue>, error out=w343:errorcluster)  [unwired: 1 in, 1 out]
      }
      event "Array CtrlCluster": Value Change {
        n246 = event-data() -> ()  [unwired: 1 in, 6 out]
        n247 = local read "Array CtrlCluster"() -> (w349:T1)
        n248 = local read "CtrlClusterOld"() -> (w350:T1)
        n249 = Not Equal?(x=w350, y=w349) -> (x != y?=w353:bool)
        n250 = case shown="True" w353 {
          frame False {
            n251 = local write "ConfChange"(FALSE ("ConfChange")) -> ()
          }
          frame True {
            n252 = local write "ConfChange"(TRUE ("ConfChange")) -> ()
          }
        }
      }
      event "Read": Value Change {
        n253 = event-data() -> ("NewVal"=w356:bool)  [unwired: 1 in, 5 out]
        n254 = case shown="True" w356 {
          frame False {
            n255 = global write "Variable global de carga.vi" "Conn"(FALSE ("Conn")) -> ()
            n256 = local write "Controllers Load"(T2 [] ("Controllers Load")) -> ()
            n257 = property on="Carga total" class="Bool (strict)"("DisabledEnum"=T3."Enabled" ("Disabled")) -> ()  [unwired: 2 in, 2 out]
            n258 = property on="Settings Nav Button" class="Bool (strict)"("DisabledEnum"=T3."Enabled" ("Disabled")) -> ()  [unwired: 2 in, 2 out]
            n259 = property on="Home Nav Button" class="Bool (strict)"("DisabledEnum"=T3."Enabled" ("Disabled")) -> ()  [unwired: 2 in, 2 out]
          }
          frame True {
            n260 = local write "Loading Text"("" ("Carga texto")) -> ()
            n261 = property on="Carga total" class="Bool (strict)"("DisabledEnum"=T3."Disabled and Grayed Out" ("Disabled")) -> ()  [unwired: 2 in, 2 out]
            n262 = property on="Settings Nav Button" class="Bool (strict)"("DisabledEnum"=T3."Disabled" ("Disabled")) -> ()  [unwired: 2 in, 2 out]
            n263 = property on="Home Nav Button" class="Bool (strict)"("DisabledEnum"=T3."Disabled" ("Disabled")) -> ()  [unwired: 2 in, 2 out]
          }
        }
      }
      event "Secret button": Value Change {
        n264 = event-data() -> ("NewVal"=w368:bool)  [unwired: 1 in, 5 out]
        n265 = case shown="False" w368 {
          frame False {
            n266 = property on="SecretAnimationCtrl" class="DigNum (strict)"("Visible"=FALSE) -> ()  [unwired: 2 in, 2 out]
          }
          frame True {
            n267 = property on="SecretAnimationCtrl" class="DigNum (strict)"("Visible"=TRUE) -> ()  [unwired: 2 in, 2 out]
          }
        }
      }
      event "SecretAnimationCtrl": Value Change {
        n268 = event-data() -> ("NewVal"=w371:i32)  [unwired: 1 in, 5 out]
        n269 = local write "Ring 2"(w371) -> ()
      }
      event "Boton Guardar Cambios": Value Change {
        n270 = event-data() -> ("NewVal"=w372:bool)  [unwired: 1 in, 5 out]
        n271 = case shown="True" w372 {
          tunnel: w376 -> [w378 w383]
          tunnel: w375 -> [w377 w381]
          tunnel: [w377 w380] -> w374
          tunnel: [w378 w379] -> w373
          frame False {
          }
          frame True {
            n272 = Enqueue Element(queue=w383, element="Guardar Cambios", error in (no error)=w381) -> (queue out=w379:refnum<queue>, error out=w380:errorcluster)  [unwired: 1 in, 1 out]
          }
        }
      }
    }
    n273 = case "guard clause" shown="No Error" w248 {
      selector: w248 -> [w249 w251]
      tunnel: w245 -> [w250 w252]
      tunnel: [w250 w254] -> w244
      tunnel: [w249 w253] -> w243
      frame No Error {
        # "No se realiza nada"
      }
      frame Error {
        # "Iniciar el proceso de Shutdown: detener el bucle del consumidor insertando el estado \"Shutdown\" al principio de la cola"
        n274 = Enqueue Element At Opposite End(queue=w252, element="Shutdown", error in (no error)=w251) -> (queue out=w254:refnum<queue>, error out=w253:errorcluster)  [unwired: 1 in, 1 out]
      }
    }
  }
  n275 = Merge Errors(w7, w11) -> (w12:errorcluster)
  n276 = Release Queue(queue=w6, error in (no error)=w12) -> (error out=w10:errorcluster)  [unwired: 1 in, 2 out]
  n277 = call <vilib>:"Simple Error Handler.vi"("error in (no error)"=w10) -> ("error out"=w4:errorcluster)  [unwired: 4 in, 4 out]
  n278 = disable-structure shown="RUN_TIME_ENGINE==True" {
    disable-tunnel: w4 -> [_ _]
    frame condition #0 {
      n279 = Quit LabVIEW() -> ()  [unwired: 1 in]
    }
    frame condition #1 (active) {
    }
  }
  "Ring 2" <- u16 0 ("Ring 2")
